vi "FlexMag - 24-03-2023.vi"() -> ()   [LabVIEW 2018] (continued)
                                n12774 = local read "ch4-3 transfer"() -> (w17942:bool)
                                n12775 = local read "ABORT"() -> (w17941:bool)
                                n12776 = Not(x=w17942) -> (.not. x?=w17940:bool)
                                n12777 = Compound Arithmetic op=OR(w17935, w17941, w17940) -> (w17939:bool)
                                }
                              }
                            }
                          }
                        }
                      }
                      frame True {
                      }
                    }
                  }
                }
              }
              frame #46 {
                n12778 = local read "ch4-3 transfer"() -> (w17949:bool)
                n12779 = case shown="True" w17949 {
                  frame False {
                  }
                  frame True {
                    n12780 = local read "ABORT"() -> (w17950:bool)
                    n12781 = case shown="False" w17950 {
                      frame False {
                        n12782 = local write "trns 4-3 led 22"(TRUE ("trns 1-2 led 1")) -> ()
                        n12783 = Wait (ms)(milliseconds to wait=u32 100) -> ()  [unwired: 1 out]
                      }
                      frame True {
                      }
                    }
                  }
                }
              }
              frame #47 {
                n12784 = local read "ch4-3 transfer"() -> (w17953:bool)
                n12785 = case shown="True" w17953 {
                  frame False {
                  }
                  frame True {
                    n12786 = local read "ABORT"() -> (w17954:bool)
                    n12787 = case shown="False" w17954 {
                      frame False {
                        n12788 = disable-structure shown="Enabled" {
                          frame Disabled {
                            n12789 = stacked-sequence {
                              frame #0 {
                                n12790 = while {
                                i -> [w17959]
                                stop <- w17960 stop-if-true
                                n12791 = Greater Or Equal?(x=w17959, y=100) -> (x >= y?=w17957:bool)
                                n12792 = case shown="True" w17957 {
                                frame False {
                                }
                                frame True {
                                n12793 = local write "Warning Message"("Transfer process canceled!\nRight Slow Sensor problem" ("Warning Message")) -> ()
                                n12794 = local write "trns error"(TRUE ("TRNS error")) -> ()
                                }
                                }
                                n12795 = local read "Cnt_Right_Slow DI"() -> (w17955:bool)
                                n12796 = case shown="True" w17955 {
                                tunnel: [TRUE ("CH1_Trns_BP_Left_DO") FALSE ("CH1_Trns_BP_Left_DO")] -> w17956
                                frame False {
                                }
                                frame True {
                                n12797 = Wait Until Next ms Multiple(millisecond multiple=u32 200) -> ()  [unwired: 1 out]
                                n12798 = local write "Cnt_Right_Slow DO"(FALSE ("TRNS error")) -> ()
                                }
                                }
                                n12799 = local read "ch4-3 transfer"() -> (w17963:bool)
                                n12800 = local read "ABORT"() -> (w17962:bool)
                                n12801 = Not(x=w17963) -> (.not. x?=w17961:bool)
                                n12802 = Compound Arithmetic op=OR(w17956, w17962, w17961) -> (w17960:bool)
                                }
                              }
                              frame #1 {
                                n12803 = while {
                                i -> [w17974]
                                stop <- w17975 stop-if-true
                                n12804 = Greater Or Equal?(x=w17974, y=100) -> (x >= y?=w17972:bool)
                                n12805 = case shown="True" w17972 {
                                frame False {
                                }
                                frame True {
                                n12806 = local write "Warning Message"("Transfer process canceled!\nRight Limit Sensor problem" ("Warning Message")) -> ()
                                n12807 = local write "trns error"(TRUE ("TRNS error")) -> ()
                                }
                                }
                                n12808 = local read "Cnt_Right_Limit DI"() -> (w17970:bool)
                                n12809 = case shown="True" w17970 {
                                tunnel: [TRUE ("CH1_Trns_BP_Left_DO") FALSE ("CH1_Trns_BP_Left_DO")] -> w17971
                                frame False {
                                }
                                frame True {
                                n12810 = Wait Until Next ms Multiple(millisecond multiple=u32 200) -> ()  [unwired: 1 out]
                                n12811 = local write "Cnt_Right_Limit DO"(FALSE ("TRNS error")) -> ()
                                }
                                }
                                n12812 = local read "ch4-3 transfer"() -> (w17978:bool)
                                n12813 = local read "ABORT"() -> (w17977:bool)
                                n12814 = Not(x=w17978) -> (.not. x?=w17976:bool)
                                n12815 = Compound Arithmetic op=OR(w17971, w17977, w17976) -> (w17975:bool)
                                }
                              }
                              frame #2 {
                                n12816 = while {
                                i -> [w17989]
                                stop <- w17990 stop-if-true
                                n12817 = Greater Or Equal?(x=w17989, y=100) -> (x >= y?=w17987:bool)
                                n12818 = case shown="True" w17987 {
                                frame False {
                                }
                                frame True {
                                n12819 = local write "Warning Message"("Transfer process canceled!\nLeft Slow Sensor problem" ("Warning Message")) -> ()
                                n12820 = local write "trns error"(TRUE ("TRNS error")) -> ()
                                }
                                }
                                n12821 = local read "Cnt_Left_Slow DI"() -> (w17985:bool)
                                n12822 = case shown="True" w17985 {
                                tunnel: [TRUE ("CH1_Trns_BP_Left_DO") FALSE ("CH1_Trns_BP_Left_DO")] -> w17986
                                frame False {
                                }
                                frame True {
                                n12823 = Wait Until Next ms Multiple(millisecond multiple=u32 200) -> ()  [unwired: 1 out]
                                n12824 = local write "Cnt_Left_Slow DO"(FALSE ("TRNS error")) -> ()
                                }
                                }
                                n12825 = local read "ch4-3 transfer"() -> (w17993:bool)
                                n12826 = local read "ABORT"() -> (w17992:bool)
                                n12827 = Not(x=w17993) -> (.not. x?=w17991:bool)
                                n12828 = Compound Arithmetic op=OR(w17986, w17992, w17991) -> (w17990:bool)
                                }
                              }
                              frame #3 {
                                n12829 = while {
                                i -> [w18004]
                                stop <- w18005 stop-if-true
                                n12830 = Greater Or Equal?(x=w18004, y=100) -> (x >= y?=w18002:bool)
                                n12831 = case shown="True" w18002 {
                                frame False {
                                }
                                frame True {
                                n12832 = local write "Warning Message"("Transfer process canceled!\nLeft Limit Sensor problem" ("Warning Message")) -> ()
                                n12833 = local write "trns error"(TRUE ("TRNS error")) -> ()
                                }
                                }
                                n12834 = local read "Cnt_Left_Limit DI"() -> (w18000:bool)
                                n12835 = case shown="True" w18000 {
                                tunnel: [TRUE ("CH1_Trns_BP_Left_DO") FALSE ("CH1_Trns_BP_Left_DO")] -> w18001
                                frame False {
                                }
                                frame True {
                                n12836 = Wait Until Next ms Multiple(millisecond multiple=u32 200) -> ()  [unwired: 1 out]
                                n12837 = local write "Cnt_Left_Limit DO"(FALSE ("TRNS error")) -> ()
                                }
                                }
                                n12838 = local read "ch4-3 transfer"() -> (w18008:bool)
                                n12839 = local read "ABORT"() -> (w18007:bool)
                                n12840 = Not(x=w18008) -> (.not. x?=w18006:bool)
                                n12841 = Compound Arithmetic op=OR(w18001, w18007, w18006) -> (w18005:bool)
                                }
                              }
                            }
                          }
                          frame Enabled {
                            w18016 = FALSE ("CH4_SRV1_Piston_For_DO")
                            w18017 = FALSE ("CH4_SRV1_Piston_For_DO")
                            n12842 = local write "CH1_Right_Limit_DO"(w18017) -> ()
                            n12843 = local write "CH1_Right_Slow_DO"(w18017) -> ()
                            n12844 = local write "CH2_Right_Limit_DO"(w18017) -> ()
                            n12845 = local write "CH2_Right_Slow_DO"(w18017) -> ()
                            n12846 = local write "CH2_Left_Slow_DO"(w18017) -> ()
                            n12847 = local write "CH2_Left_Limit_DO"(w18017) -> ()
                            n12848 = Wait (ms)(milliseconds to wait=u32 2000) -> ()  [unwired: 1 out]
                            n12849 = local write "CH3_Right_Limit_DO"(w18016) -> ()
                            n12850 = local write "CH3_Right_Slow_DO"(w18016) -> ()
                            n12851 = local write "CH3_Left_Slow_DO"(w18016) -> ()
                            n12852 = local write "CH3_Left_Limit_DO"(w18016) -> ()
                            n12853 = local write "CH4_Left_Limit_DO"(w18016) -> ()
                            n12854 = local write "CH4_Left_Slow_DO"(w18016) -> ()
                          }
                        }
                      }
                      frame True {
                      }
                    }
                  }
                }
              }
              frame #48 {
                n12855 = local read "ch4-3 transfer"() -> (w18018:bool)
                n12856 = case shown="True" w18018 {
                  frame False {
                  }
                  frame True {
                    n12857 = local read "ABORT"() -> (w18019:bool)
                    n12858 = case shown="False" w18019 {
                      frame False {
                        n12859 = local write "trns 4-3 led 23"(TRUE ("trns 1-2 led 17")) -> ()
                        n12860 = Wait (ms)(milliseconds to wait=u32 100) -> ()  [unwired: 1 out]
                      }
                      frame True {
                      }
                    }
                  }
                }
              }
              frame #49 {
                n12861 = local read "ch4-3 transfer"() -> (w18022:bool)
                n12862 = case shown="True" w18022 {
                  frame False {
                  }
                  frame True {
                    n12863 = local read "ABORT"() -> (w18023:bool)
                    n12864 = case shown="False" w18023 {
                      frame False {
                        n12865 = local write "Buzzer DO"(TRUE ("trns 1-2 led 17")) -> ()
                        n12866 = Wait (ms)(milliseconds to wait=u32 3000) -> ()  [unwired: 1 out]
                        n12867 = local write "System Status"("CH4 to CH3  Transfer Completed" ("System Status")) -> ()
                      }
                      frame True {
                      }
                    }
                  }
                }
              }
              frame #50 {
                n12868 = local read "ch4-3 transfer"() -> (w18027:bool)
                n12869 = case shown="True" w18027 {
                  frame False {
                  }
                  frame True {
                    n12870 = local read "ABORT"() -> (w18028:bool)
                    n12871 = case shown="False" w18028 {
                      frame False {
                        w18029 = u16 3 items=["CH1"=1, "CH2"=2, "CH3"=3, "CH4"=4] ("cassette position selection")
                        w18030 = FALSE ("trns 1-2 led 17")
                        n12872 = Wait (ms)(milliseconds to wait=u32 1000) -> ()  [unwired: 1 out]
                        n12873 = local write "ch4-3 transfer"(FALSE ("trns 1-2 led 17")) -> ()
                        n12874 = local write "Buzzer DO"(FALSE ("trns 1-2 led 17")) -> ()
                        n12875 = local write "cassette position selection"(w18029) -> ()
                        n12876 = local write "System Status"("SEMI-AUTOMATIC MODE " ("System Status")) -> ()
                        n12877 = Not(x=w18030) -> (.not. x?=w18031:bool)
                        n12878 = local write "present location"(3.0 ("present location")) -> ()
                        n12879 = local write "casette_ch1_gui"(w18030) -> ()
                        n12880 = local write "casette_ch2_gui"(w18030) -> ()
                        n12881 = local write "casette_ch3_gui"(w18031) -> ()
                        n12882 = local write "casette_ch4_gui"(w18030) -> ()
                      }
                      frame True {
                      }
                    }
                  }
                }
              }
              frame #51 {
              }
            }
          }
          frame True {
          }
        }
      }
    }
  }
  n12883 = while {
    stop <- FALSE stop-if-true
    n12884 = Wait Until Next ms Multiple(millisecond multiple=u32 300) -> ()  [unwired: 1 out]
    n12885 = case shown="True" "trns pre check" {
      frame False {
      }
      frame True {
        n12886 = stacked-sequence {
          frame #0 {
            n12887 = flat-sequence {
              frame #0 {
                n12888 = local write "trns clear"(TRUE ("trns clear")) -> ()
              }
              frame #1 {
                n12889 = Wait (ms)(milliseconds to wait=u32 1000) -> ()  [unwired: 1 out]
              }
            }
          }
          frame #1 {
            n12890 = local read "ABORT"() -> (w18042:bool)
            n12891 = case shown="False" w18042 {
              frame False {
                n12892 = local read "trns pre check"() -> (w18043:bool)
                n12893 = case shown="True" w18043 {
                  frame False {
                  }
                  frame True {
                    n12894 = while {
                      i -> [w18050]
                      stop <- w18047 stop-if-true
                      n12895 = Greater Or Equal?(x=w18050, y=600) -> (x >= y?=w18048:bool)
                      n12896 = case shown="True" w18048 {
                        frame False {
                        }
                        frame True {
                          n12897 = local write "Warning Message"("Transfer process canceled!\nCH1 srv piston problem" ("Warning Message")) -> ()
                          n12898 = local write "trns error"(TRUE ("TRNS error")) -> ()
                        }
                      }
                      n12899 = local read "CH1_SRV1_Piston_Back_DI"() -> (w18052:bool)
                      n12900 = case shown="True" w18052 {
                        tunnel: [FALSE TRUE] -> w18051
                        frame False {
                          n12901 = local write "CH1_SRV1_Piston_Back_DO"(TRUE ("CH1_SRV1_Piston_Back_DO")) -> ()
                          n12902 = local write "CH1_SRV1_Piston_For_DO"(FALSE ("CH1_SRV1_Piston_For_DO")) -> ()
                          n12903 = Wait Until Next ms Multiple(millisecond multiple=u32 200) -> ()  [unwired: 1 out]
                        }
                        frame True {
                        }
                      }
                      n12904 = local read "trns pre check"() -> (w18044:bool)
                      n12905 = local read "ABORT"() -> (w18046:bool)
                      n12906 = Not(x=w18044) -> (.not. x?=w18045:bool)
                      n12907 = Compound Arithmetic op=OR(w18051, w18046, w18045) -> (w18047:bool)
                    }
                  }
                }
              }
              frame True {
              }
            }
          }
          frame #2 {
            n12908 = local read "trns pre check"() -> (w18060:bool)
            n12909 = case shown="True" w18060 {
              frame False {
              }
              frame True {
                n12910 = local read "ABORT"() -> (w18061:bool)
                n12911 = case shown="False" w18061 {
                  frame False {
                    n12912 = local write "trns pre check led 1"(TRUE ("1")) -> ()
                    n12913 = Wait (ms)(milliseconds to wait=u32 100) -> ()  [unwired: 1 out]
                  }
                  frame True {
                  }
                }
              }
            }
          }
          frame #3 {
            n12914 = local read "ABORT"() -> (w18064:bool)
            n12915 = case shown="False" w18064 {
              frame False {
                n12916 = local read "trns pre check"() -> (w18065:bool)
                n12917 = case shown="True" w18065 {
                  frame False {
                  }
                  frame True {
                    n12918 = while {
                      i -> [w18072]
                      stop <- w18069 stop-if-true
                      n12919 = Greater Or Equal?(x=w18072, y=600) -> (x >= y?=w18070:bool)
                      n12920 = case shown="True" w18070 {
                        frame False {
                        }
                        frame True {
                          n12921 = local write "Warning Message"("Transfer process canceled!\nCH2 srv piston problem" ("Warning Message")) -> ()
                          n12922 = local write "trns error"(TRUE ("TRNS error")) -> ()
                        }
                      }
                      n12923 = local read "CH2_SRV1_Piston_Back_DI"() -> (w18074:bool)
                      n12924 = case shown="False" w18074 {
                        tunnel: [FALSE TRUE] -> w18073
                        frame False {
                          n12925 = local write "CH2_SRV1_Piston_Back_DO"(TRUE ("CH1_SRV1_Piston_Back_DO")) -> ()
                          n12926 = local write "CH2_SRV1_Piston_For_DO"(FALSE ("CH2_SRV1_Piston_For_DO")) -> ()
                          n12927 = Wait Until Next ms Multiple(millisecond multiple=u32 200) -> ()  [unwired: 1 out]
                        }
                        frame True {
                        }
                      }
                      n12928 = local read "trns pre check"() -> (w18066:bool)
                      n12929 = local read "ABORT"() -> (w18068:bool)
                      n12930 = Not(x=w18066) -> (.not. x?=w18067:bool)
                      n12931 = Compound Arithmetic op=OR(w18073, w18068, w18067) -> (w18069:bool)
                    }
                  }
                }
              }
              frame True {
              }
            }
          }
          frame #4 {
            n12932 = local read "trns pre check"() -> (w18082:bool)
            n12933 = case shown="True" w18082 {
              frame False {
              }
              frame True {
                n12934 = local read "ABORT"() -> (w18083:bool)
                n12935 = case shown="False" w18083 {
                  frame False {
                    n12936 = local write "trns pre check led 2"(TRUE ("1")) -> ()
                    n12937 = Wait (ms)(milliseconds to wait=u32 100) -> ()  [unwired: 1 out]
                  }
                  frame True {
                  }
                }
              }
            }
          }
          frame #5 {
            n12938 = local read "ABORT"() -> (w18086:bool)
            n12939 = case shown="False" w18086 {
              frame False {
                n12940 = local read "trns pre check"() -> (w18087:bool)
                n12941 = case shown="True" w18087 {
                  frame False {
                  }
                  frame True {
                    n12942 = while {
                      i -> [w18094]
                      stop <- w18091 stop-if-true
                      n12943 = Greater Or Equal?(x=w18094, y=600) -> (x >= y?=w18092:bool)
                      n12944 = case shown="True" w18092 {
                        frame False {
                        }
                        frame True {
                          n12945 = local write "Warning Message"("Transfer process canceled!\nCH3 srv piston problem" ("Warning Message")) -> ()
                          n12946 = local write "trns error"(TRUE ("TRNS error")) -> ()
                        }
                      }
                      n12947 = local read "CH3_SRV1_Piston_Back_DI"() -> (w18096:bool)
                      n12948 = case shown="False" w18096 {
                        tunnel: [FALSE TRUE] -> w18095
                        frame False {
                          n12949 = local write "CH3_SRV1_Piston_Back_DO"(TRUE ("CH1_SRV1_Piston_Back_DO")) -> ()
                          n12950 = local write "CH3_SRV1_Piston_For_DO"(FALSE ("CH3_SRV1_Piston_For_DO")) -> ()
                          n12951 = Wait Until Next ms Multiple(millisecond multiple=u32 200) -> ()  [unwired: 1 out]
                        }
                        frame True {
                        }
                      }
                      n12952 = local read "trns pre check"() -> (w18088:bool)
                      n12953 = local read "ABORT"() -> (w18090:bool)
                      n12954 = Not(x=w18088) -> (.not. x?=w18089:bool)
                      n12955 = Compound Arithmetic op=OR(w18095, w18090, w18089) -> (w18091:bool)
                    }
                  }
                }
              }
              frame True {
              }
            }
          }
          frame #6 {
            n12956 = local read "trns pre check"() -> (w18104:bool)
            n12957 = case shown="True" w18104 {
              frame False {
              }
              frame True {
                n12958 = local read "ABORT"() -> (w18105:bool)
                n12959 = case shown="False" w18105 {
                  frame False {
                    n12960 = local write "trns pre check led 3"(TRUE ("1")) -> ()
                    n12961 = Wait (ms)(milliseconds to wait=u32 100) -> ()  [unwired: 1 out]
                  }
                  frame True {
                  }
                }
              }
            }
          }
          frame #7 {
            n12962 = local read "ABORT"() -> (w18108:bool)
            n12963 = case shown="False" w18108 {
              frame False {
                n12964 = local read "trns pre check"() -> (w18109:bool)
                n12965 = case shown="True" w18109 {
                  frame False {
                  }
                  frame True {
                    n12966 = while {
                      i -> [w18116]
                      stop <- w18113 stop-if-true
                      n12967 = Greater Or Equal?(x=w18116, y=600) -> (x >= y?=w18114:bool)
                      n12968 = case shown="True" w18114 {
                        frame False {
                        }
                        frame True {
                          n12969 = local write "Warning Message"("Transfer process canceled!\nCH4 srv piston problem" ("Warning Message")) -> ()
                          n12970 = local write "trns error"(TRUE ("TRNS error")) -> ()
                        }
                      }
                      n12971 = local read "CH4_SRV1_Piston_Back_DI"() -> (w18118:bool)
                      n12972 = case shown="False" w18118 {
                        tunnel: [FALSE TRUE] -> w18117
                        frame False {
                          n12973 = local write "CH4_SRV1_Piston_Back_DO"(TRUE ("CH1_SRV1_Piston_Back_DO")) -> ()
                          n12974 = local write "CH4_SRV1_Piston_For_DO"(FALSE ("CH4_SRV1_Piston_For_DO")) -> ()
                          n12975 = Wait Until Next ms Multiple(millisecond multiple=u32 200) -> ()  [unwired: 1 out]
                        }
                        frame True {
                        }
                      }
                      n12976 = local read "trns pre check"() -> (w18110:bool)
                      n12977 = local read "ABORT"() -> (w18112:bool)
                      n12978 = Not(x=w18110) -> (.not. x?=w18111:bool)
                      n12979 = Compound Arithmetic op=OR(w18117, w18112, w18111) -> (w18113:bool)
                    }
                  }
                }
              }
              frame True {
              }
            }
          }
          frame #8 {
            n12980 = local read "trns pre check"() -> (w18126:bool)
            n12981 = case shown="True" w18126 {
              frame False {
              }
              frame True {
                n12982 = local read "ABORT"() -> (w18127:bool)
                n12983 = case shown="False" w18127 {
                  frame False {
                    n12984 = local write "trns pre check led 4"(TRUE ("1")) -> ()
                    n12985 = Wait (ms)(milliseconds to wait=u32 100) -> ()  [unwired: 1 out]
                  }
                  frame True {
                  }
                }
              }
            }
          }
          frame #9 {
            n12986 = local read "ABORT"() -> (w18130:bool)
            n12987 = case shown="False" w18130 {
              frame False {
                n12988 = local read "trns pre check"() -> (w18131:bool)
                n12989 = case shown="True" w18131 {
                  frame False {
                  }
                  frame True {
                    n12990 = while {
                      i -> [w18138]
                      stop <- w18135 stop-if-true
                      n12991 = Greater Or Equal?(x=w18138, y=600) -> (x >= y?=w18136:bool)
                      n12992 = case shown="True" w18136 {
                        frame False {
                        }
                        frame True {
                          n12993 = local write "Warning Message"("Transfer process canceled!\nCH1 PetCool problem" ("Warning Message")) -> ()
                          n12994 = local write "trns error"(TRUE ("TRNS error")) -> ()
                        }
                      }
                      n12995 = local read "CH1_PetCool_Up_DI"() -> (w18140:bool)
                      n12996 = case shown="False" w18140 {
                        tunnel: [FALSE TRUE] -> w18139
                        frame False {
                          n12997 = local write "CH1_PetCool_Down_DO"(FALSE ("CH4_SRV1_Piston_For_DO")) -> ()
                          n12998 = local write "CH1_PetCool_Up_DO"(TRUE ("CH1_SRV1_Piston_Back_DO")) -> ()
                          n12999 = Wait Until Next ms Multiple(millisecond multiple=u32 200) -> ()  [unwired: 1 out]
                        }
                        frame True {
                        }
                      }
                      n13000 = local read "trns pre check"() -> (w18132:bool)
                      n13001 = local read "ABORT"() -> (w18134:bool)
                      n13002 = Not(x=w18132) -> (.not. x?=w18133:bool)
                      n13003 = Compound Arithmetic op=OR(w18139, w18134, w18133) -> (w18135:bool)
                    }
                  }
                }
              }
              frame True {
              }
            }
          }
          frame #10 {
            n13004 = local read "trns pre check"() -> (w18148:bool)
            n13005 = case shown="True" w18148 {
              frame False {
              }
              frame True {
                n13006 = local read "ABORT"() -> (w18149:bool)
                n13007 = case shown="False" w18149 {
                  frame False {
                    n13008 = local write "trns pre check led 5"(TRUE ("1")) -> ()
                    n13009 = Wait (ms)(milliseconds to wait=u32 100) -> ()  [unwired: 1 out]
                  }
                  frame True {
                  }
                }
              }
            }
          }
          frame #11 {
            n13010 = local read "ABORT"() -> (w18152:bool)
            n13011 = case shown="False" w18152 {
              frame False {
                n13012 = local read "trns pre check"() -> (w18153:bool)
                n13013 = case shown="True" w18153 {
                  frame False {
                  }
                  frame True {
                    n13014 = while {
                      i -> [w18160]
                      stop <- w18157 stop-if-true
                      n13015 = Greater Or Equal?(x=w18160, y=600) -> (x >= y?=w18158:bool)
                      n13016 = case shown="True" w18158 {
                        frame False {
                        }
                        frame True {
                          n13017 = local write "Warning Message"("Transfer process canceled!\nCH2 PetCool problem" ("Warning Message")) -> ()
                          n13018 = local write "trns error"(TRUE ("TRNS error")) -> ()
                        }
                      }
                      n13019 = local read "CH2_PetCool_Up_DI"() -> (w18162:bool)
                      n13020 = case shown="False" w18162 {
                        tunnel: [FALSE TRUE] -> w18161
                        frame False {
                          n13021 = local write "CH2_PetCool_Down_DO"(FALSE ("CH4_SRV1_Piston_For_DO")) -> ()
                          n13022 = local write "CH2_PetCool_Up_DO"(TRUE ("CH1_SRV1_Piston_Back_DO")) -> ()
                          n13023 = Wait Until Next ms Multiple(millisecond multiple=u32 200) -> ()  [unwired: 1 out]
                        }
                        frame True {
                        }
                      }
                      n13024 = local read "trns pre check"() -> (w18154:bool)
                      n13025 = local read "ABORT"() -> (w18156:bool)
                      n13026 = Not(x=w18154) -> (.not. x?=w18155:bool)
                      n13027 = Compound Arithmetic op=OR(w18161, w18156, w18155) -> (w18157:bool)
                    }
                  }
                }
              }
              frame True {
              }
            }
          }
          frame #12 {
            n13028 = local read "trns pre check"() -> (w18170:bool)
            n13029 = case shown="True" w18170 {
              frame False {
              }
              frame True {
                n13030 = local read "ABORT"() -> (w18171:bool)
                n13031 = case shown="False" w18171 {
                  frame False {
                    n13032 = local write "trns pre check led 6"(TRUE ("1")) -> ()
                    n13033 = Wait (ms)(milliseconds to wait=u32 100) -> ()  [unwired: 1 out]
                  }
                  frame True {
                  }
                }
              }
            }
          }
          frame #13 {
            n13034 = local read "ABORT"() -> (w18174:bool)
            n13035 = case shown="False" w18174 {
              frame False {
                n13036 = local read "trns pre check"() -> (w18175:bool)
                n13037 = case shown="True" w18175 {
                  frame False {
                  }
                  frame True {
                    n13038 = while {
                      i -> [w18182]
                      stop <- w18179 stop-if-true
                      n13039 = Greater Or Equal?(x=w18182, y=600) -> (x >= y?=w18180:bool)
                      n13040 = case shown="True" w18180 {
                        frame False {
                        }
                        frame True {
                          n13041 = local write "Warning Message"("Transfer process canceled!\nCH3 PetCool problem" ("Warning Message")) -> ()
                          n13042 = local write "trns error"(TRUE ("TRNS error")) -> ()
                        }
                      }
                      n13043 = local read "CH3_PetCool_Up_DI"() -> (w18184:bool)
                      n13044 = case shown="False" w18184 {
                        tunnel: [FALSE TRUE] -> w18183
                        frame False {
                          n13045 = local write "CH3_PetCool_Down_DO"(FALSE ("CH4_SRV1_Piston_For_DO")) -> ()
                          n13046 = local write "CH3_PetCool_Up_DO"(TRUE ("CH1_SRV1_Piston_Back_DO")) -> ()
                          n13047 = Wait Until Next ms Multiple(millisecond multiple=u32 200) -> ()  [unwired: 1 out]
                        }
                        frame True {
                        }
                      }
                      n13048 = local read "trns pre check"() -> (w18176:bool)
                      n13049 = local read "ABORT"() -> (w18178:bool)
                      n13050 = Not(x=w18176) -> (.not. x?=w18177:bool)
                      n13051 = Compound Arithmetic op=OR(w18183, w18178, w18177) -> (w18179:bool)
                    }
                  }
                }
              }
              frame True {
              }
            }
          }
          frame #14 {
            n13052 = local read "trns pre check"() -> (w18192:bool)
            n13053 = case shown="True" w18192 {
              frame False {
              }
              frame True {
                n13054 = local read "ABORT"() -> (w18193:bool)
                n13055 = case shown="False" w18193 {
                  frame False {
                    n13056 = local write "trns pre check led 7"(TRUE ("1")) -> ()
                    n13057 = Wait (ms)(milliseconds to wait=u32 100) -> ()  [unwired: 1 out]
                  }
                  frame True {
                  }
                }
              }
            }
          }
          frame #15 {
            n13058 = local read "ABORT"() -> (w18196:bool)
            n13059 = case shown="False" w18196 {
              frame False {
                n13060 = local read "trns pre check"() -> (w18197:bool)
                n13061 = case shown="True" w18197 {
                  frame False {
                  }
                  frame True {
                    n13062 = while {
                      i -> [w18204]
                      stop <- w18201 stop-if-true
                      n13063 = Greater Or Equal?(x=w18204, y=600) -> (x >= y?=w18202:bool)
                      n13064 = case shown="True" w18202 {
                        frame False {
                        }
                        frame True {
                          n13065 = local write "Warning Message"("Transfer process canceled!\nCH4 PetCool problem" ("Warning Message")) -> ()
                          n13066 = local write "trns error"(TRUE ("TRNS error")) -> ()
                        }
                      }
                      n13067 = local read "CH4_PetCool_Up_DI"() -> (w18206:bool)
                      n13068 = case shown="False" w18206 {
                        tunnel: [FALSE TRUE] -> w18205
                        frame False {
                          n13069 = local write "CH4_PetCool_Down_DO"(FALSE ("CH4_SRV1_Piston_For_DO")) -> ()
                          n13070 = local write "CH4_PetCool_Up_DO"(TRUE ("CH1_SRV1_Piston_Back_DO")) -> ()
                          n13071 = Wait Until Next ms Multiple(millisecond multiple=u32 200) -> ()  [unwired: 1 out]
                        }
                        frame True {
                        }
                      }
                      n13072 = local read "trns pre check"() -> (w18198:bool)
                      n13073 = local read "ABORT"() -> (w18200:bool)
                      n13074 = Not(x=w18198) -> (.not. x?=w18199:bool)
                      n13075 = Compound Arithmetic op=OR(w18205, w18200, w18199) -> (w18201:bool)
                    }
                  }
                }
              }
              frame True {
              }
            }
          }
          frame #16 {
            n13076 = local read "trns pre check"() -> (w18214:bool)
            n13077 = case shown="True" w18214 {
              frame False {
              }
              frame True {
                n13078 = local read "ABORT"() -> (w18215:bool)
                n13079 = case shown="False" w18215 {
                  frame False {
                    n13080 = local write "trns pre check led 8"(TRUE ("1")) -> ()
                    n13081 = Wait (ms)(milliseconds to wait=u32 100) -> ()  [unwired: 1 out]
                  }
                  frame True {
                  }
                }
              }
            }
          }
          frame #17 {
            n13082 = local read "ABORT"() -> (w18218:bool)
            n13083 = case shown="False" w18218 {
              frame False {
                n13084 = local read "trns pre check"() -> (w18219:bool)
                n13085 = case shown="True" w18219 {
                  frame False {
                  }
                  frame True {
                    n13086 = while {
                      i -> [w18226]
                      stop <- w18223 stop-if-true
                      n13087 = Greater Or Equal?(x=w18226, y=600) -> (x >= y?=w18224:bool)
                      n13088 = case shown="True" w18224 {
                        frame False {
                        }
                        frame True {
                          n13089 = local write "Warning Message"("Transfer process canceled!\nCH1 Cassette Fix problem" ("Warning Message")) -> ()
                          n13090 = local write "trns error"(TRUE ("TRNS error")) -> ()
                        }
                      }
                      n13091 = local read "CH1_Cst_Fix_Up_DI"() -> (w18228:bool)
                      n13092 = case shown="False" w18228 {
                        tunnel: [FALSE TRUE] -> w18227
                        frame False {
                          n13093 = local write "CH1_Cst_Fix_DO"(FALSE ("CH1_SRV1_Piston_Back_DO")) -> ()
                          n13094 = Wait Until Next ms Multiple(millisecond multiple=u32 200) -> ()  [unwired: 1 out]
                        }
                        frame True {
                        }
                      }
                      n13095 = local read "trns pre check"() -> (w18220:bool)
                      n13096 = local read "ABORT"() -> (w18222:bool)
                      n13097 = Not(x=w18220) -> (.not. x?=w18221:bool)
                      n13098 = Compound Arithmetic op=OR(w18227, w18222, w18221) -> (w18223:bool)
                    }
                  }
                }
              }
              frame True {
              }
            }
          }
          frame #18 {
            n13099 = local read "trns pre check"() -> (w18235:bool)
            n13100 = case shown="True" w18235 {
              frame False {
              }
              frame True {
                n13101 = local read "ABORT"() -> (w18236:bool)
                n13102 = case shown="False" w18236 {
                  frame False {
                    n13103 = local write "trns pre check led 9"(TRUE ("1")) -> ()
                    n13104 = Wait (ms)(milliseconds to wait=u32 100) -> ()  [unwired: 1 out]
                  }
                  frame True {
                  }
                }
              }
            }
          }
          frame #19 {
            n13105 = local read "ABORT"() -> (w18239:bool)
            n13106 = case shown="False" w18239 {
              frame False {
                n13107 = local read "trns pre check"() -> (w18240:bool)
                n13108 = case shown="True" w18240 {
                  frame False {
                  }
                  frame True {
                    n13109 = while {
                      i -> [w18247]
                      stop <- w18244 stop-if-true
                      n13110 = Greater Or Equal?(x=w18247, y=600) -> (x >= y?=w18245:bool)
                      n13111 = case shown="True" w18245 {
                        frame False {
                        }
                        frame True {
                          n13112 = local write "Warning Message"("Transfer process canceled!\nCH2 Cassette Fix problem" ("Warning Message")) -> ()
                          n13113 = local write "trns error"(TRUE ("TRNS error")) -> ()
                        }
                      }
                      n13114 = local read "CH2_Cst_Fix_Up_DI"() -> (w18249:bool)
                      n13115 = case shown="False" w18249 {
                        tunnel: [FALSE TRUE] -> w18248
                        frame False {
                          n13116 = local write "CH2_Cst_Fix_DO"(FALSE ("CH1_SRV1_Piston_Back_DO")) -> ()
                          n13117 = Wait Until Next ms Multiple(millisecond multiple=u32 200) -> ()  [unwired: 1 out]
                        }
                        frame True {
                        }
                      }
                      n13118 = local read "trns pre check"() -> (w18241:bool)
                      n13119 = local read "ABORT"() -> (w18243:bool)
                      n13120 = Not(x=w18241) -> (.not. x?=w18242:bool)
                      n13121 = Compound Arithmetic op=OR(w18248, w18243, w18242) -> (w18244:bool)
                    }
                  }
                }
              }
              frame True {
              }
            }
          }
          frame #20 {
            n13122 = local read "trns pre check"() -> (w18256:bool)
            n13123 = case shown="True" w18256 {
              frame False {
              }
              frame True {
                n13124 = local read "ABORT"() -> (w18257:bool)
                n13125 = case shown="False" w18257 {
                  frame False {
                    n13126 = local write "trns pre check led 10"(TRUE ("1")) -> ()
                    n13127 = Wait (ms)(milliseconds to wait=u32 100) -> ()  [unwired: 1 out]
                  }
                  frame True {
                  }
                }
              }
            }
          }
          frame #21 {
            n13128 = local read "ABORT"() -> (w18260:bool)
            n13129 = case shown="False" w18260 {
              frame False {
                n13130 = local read "trns pre check"() -> (w18261:bool)
                n13131 = case shown="True" w18261 {
                  frame False {
                  }
                  frame True {
                    n13132 = while {
                      i -> [w18268]
                      stop <- w18265 stop-if-true
                      n13133 = Greater Or Equal?(x=w18268, y=600) -> (x >= y?=w18266:bool)
                      n13134 = case shown="True" w18266 {
                        frame False {
                        }
                        frame True {
                          n13135 = local write "Warning Message"("Transfer process canceled!\nCH3 Cassette Fix problem" ("Warning Message")) -> ()
                          n13136 = local write "trns error"(TRUE ("TRNS error")) -> ()
                        }
                      }
                      n13137 = local read "CH3_Cst_Fix_Up_DI"() -> (w18270:bool)
                      n13138 = case shown="False" w18270 {
                        tunnel: [FALSE TRUE] -> w18269
                        frame False {
                          n13139 = local write "CH3_Cst_Fix_DO"(FALSE ("CH1_SRV1_Piston_Back_DO")) -> ()
                          n13140 = Wait Until Next ms Multiple(millisecond multiple=u32 200) -> ()  [unwired: 1 out]
                        }
                        frame True {
                        }
                      }
                      n13141 = local read "trns pre check"() -> (w18262:bool)
                      n13142 = local read "ABORT"() -> (w18264:bool)
                      n13143 = Not(x=w18262) -> (.not. x?=w18263:bool)
                      n13144 = Compound Arithmetic op=OR(w18269, w18264, w18263) -> (w18265:bool)
                    }
                  }
                }
              }
              frame True {
              }
            }
          }
          frame #22 {
            n13145 = local read "trns pre check"() -> (w18277:bool)
            n13146 = case shown="True" w18277 {
              frame False {
              }
              frame True {
                n13147 = local read "ABORT"() -> (w18278:bool)
                n13148 = case shown="False" w18278 {
                  frame False {
                    n13149 = local write "trns pre check led 11"(TRUE ("1")) -> ()
                    n13150 = Wait (ms)(milliseconds to wait=u32 100) -> ()  [unwired: 1 out]
                  }
                  frame True {
                  }
                }
              }
            }
          }
          frame #23 {
            n13151 = local read "ABORT"() -> (w18281:bool)
            n13152 = case shown="False" w18281 {
              frame False {
                n13153 = local read "trns pre check"() -> (w18282:bool)
                n13154 = case shown="True" w18282 {
                  frame False {
                  }
                  frame True {
                    n13155 = while {
                      i -> [w18289]
                      stop <- w18286 stop-if-true
                      n13156 = Greater Or Equal?(x=w18289, y=600) -> (x >= y?=w18287:bool)
                      n13157 = case shown="True" w18287 {
                        frame False {
                        }
                        frame True {
                          n13158 = local write "Warning Message"("Transfer process canceled!\nCH4 Cassette Fix problem" ("Warning Message")) -> ()
                          n13159 = local write "trns error"(TRUE ("TRNS error")) -> ()
                        }
                      }
                      n13160 = local read "CH4_Cst_Fix_Up_DI"() -> (w18291:bool)
                      n13161 = case shown="False" w18291 {
                        tunnel: [FALSE TRUE] -> w18290
                        frame False {
                          n13162 = local write "CH4_Cst_Fix_DO"(FALSE ("CH1_SRV1_Piston_Back_DO")) -> ()
                          n13163 = Wait Until Next ms Multiple(millisecond multiple=u32 200) -> ()  [unwired: 1 out]
                        }
                        frame True {
                        }
                      }
                      n13164 = local read "trns pre check"() -> (w18283:bool)
                      n13165 = local read "ABORT"() -> (w18285:bool)
                      n13166 = Not(x=w18283) -> (.not. x?=w18284:bool)
                      n13167 = Compound Arithmetic op=OR(w18290, w18285, w18284) -> (w18286:bool)
                    }
                  }
                }
              }
              frame True {
              }
            }
          }
          frame #24 {
            n13168 = local read "trns pre check"() -> (w18298:bool)
            n13169 = case shown="True" w18298 {
              frame False {
              }
              frame True {
                n13170 = local read "ABORT"() -> (w18299:bool)
                n13171 = case shown="False" w18299 {
                  frame False {
                    n13172 = local write "trns pre check led 12"(TRUE ("1")) -> ()
                    n13173 = Wait (ms)(milliseconds to wait=u32 100) -> ()  [unwired: 1 out]
                  }
                  frame True {
                  }
                }
              }
            }
          }
          frame #25 {
            n13174 = local read "trns pre check"() -> (w18302:bool)
            n13175 = case shown="True" w18302 {
              frame False {
              }
              frame True {
                n13176 = local read "ABORT"() -> (w18303:bool)
                n13177 = case shown="False" w18303 {
                  frame False {
                    n13178 = local write "trns pre check"(FALSE ("trns pre check")) -> ()
                    n13179 = Wait (ms)(milliseconds to wait=u32 100) -> ()  [unwired: 1 out]
                  }
                  frame True {
                  }
                }
              }
            }
          }
        }
      }
    }
  }
  n13180 = while {
    stop <- FALSE stop-if-true
    n13181 = local read "ABORT"() -> (w18307:bool)
    n13182 = Wait Until Next ms Multiple(millisecond multiple=u32 300) -> ()  [unwired: 1 out]
    n13183 = case shown="True" "TC parameter set" {
      tunnel: w18307 -> [_ w18314]
      tunnel: "Roll Forw" -> [_ w18313]
      frame False {
        "parameters led" <- FALSE
      }
      frame True {
        n13184 = case shown="False" w18314 {
          tunnel: w18313 -> [w18315 _]
          frame False {
            n13185 = case shown="True" w18315 {
              frame False {
                n13186 = stacked-sequence {
                  frame #0 {
                    n13187 = local write "TC1_close_loop_coefficient"(sgl 0.0 ("TC1_close_loop_coefficient")) -> ()
                    n13188 = local write "TC1_speed_coefficient_value"(sgl 100.0 ("TC1_speed_coefficient_value")) -> ()
                    n13189 = local write "TC1_AO1_upper_limit_value"(sgl 10.0 ("TC1_speed_coefficient_value")) -> ()
                    n13190 = local write "TC1_regulation_type_value"(sgl 0.0 ("TC1_speed_coefficient_value")) -> ()
                    n13191 = local write "TC1_AO1_bottom_limit_value"(sgl 0.0 ("TC1_speed_coefficient_value")) -> ()
                    n13192 = local write "TC1_setpoint_type_value"(sgl 0.0 ("TC1_speed_coefficient_value")) -> ()
                    n13193 = Wait (ms)(milliseconds to wait=u32 100) -> ()  [unwired: 1 out]
                    n13194 = local write "TC1_speed_gain_value"(sgl 0.0 ("TC1_speed_gain_value")) -> ()
                    n13195 = local write "TC2_close_loop_coefficient"(sgl 100.0 ("TC2_close_loop_coefficient")) -> ()
                    n13196 = local write "TC2_speed_coefficient_value"(sgl 0.0 ("TC2_speed_coefficient_value")) -> ()
                    n13197 = local write "TC2_AO1_upper_limit_value"(sgl 10.0 ("TC2_speed_gain_value")) -> ()
                    n13198 = local write "TC2_regulation_type_value"(sgl 1.0 ("TC2_speed_coefficient_value")) -> ()
                    n13199 = local write "TC2_speed_gain_value"(sgl 0.0 ("TC2_speed_gain_value")) -> ()
                    n13200 = local write "TC2_AO1_bottom_limit_value"(sgl 0.0 ("TC2_speed_coefficient_value")) -> ()
                    n13201 = local write "TC2_setpoint_type_value"(sgl 0.0 ("TC2_speed_coefficient_value")) -> ()
                  }
                  frame #1 {
                    n13202 = local write "TC1_close_loop_set"(TRUE ("TC1_close_loop_set")) -> ()
                  }
                  frame #2 {
                    n13203 = flat-sequence {
                      frame #0 {
                        n13204 = local read "waiting_TC"() -> (w18332:u32)
                        n13205 = Wait (ms)(milliseconds to wait=w18332) -> ()  [unwired: 1 out]
                      }
                      frame #1 {
                        n13206 = while {
                          stop <- w18333 stop-if-true
                          n13207 = local read "TC1_close_loop_set"() -> (w18334:bool)
                          n13208 = Wait Until Next ms Multiple(millisecond multiple=u32 300) -> ()  [unwired: 1 out]
                          n13209 = Not(x=w18334) -> (.not. x?=w18333:bool)
                        }
                      }
                    }
                  }
                  frame #3 {
                    n13210 = local write "TC1_speed_gain_set"(TRUE ("TC1_close_loop_set")) -> ()
                  }
                  frame #4 {
                    n13211 = flat-sequence {
                      frame #0 {
                        n13212 = local read "waiting_TC"() -> (w18337:u32)
                        n13213 = Wait (ms)(milliseconds to wait=w18337) -> ()  [unwired: 1 out]
                      }
                      frame #1 {
                        n13214 = while {
                          stop <- w18339 stop-if-true
                          n13215 = local read "TC1_speed_gain_set"() -> (w18338:bool)
                          n13216 = Wait Until Next ms Multiple(millisecond multiple=u32 300) -> ()  [unwired: 1 out]
                          n13217 = Not(x=w18338) -> (.not. x?=w18339:bool)
                        }
                      }
                    }
                  }
                  frame #5 {
                    n13218 = local write "TC1_speed_coefficient_set"(TRUE ("TC1_close_loop_set")) -> ()
                  }
                  frame #6 {
                    n13219 = flat-sequence {
                      frame #0 {
                        n13220 = local read "waiting_TC"() -> (w18342:u32)
                        n13221 = Wait (ms)(milliseconds to wait=w18342) -> ()  [unwired: 1 out]
                      }
                      frame #1 {
                        n13222 = while {
                          stop <- w18343 stop-if-true
                          n13223 = local read "TC1_speed_coefficient_set"() -> (w18344:bool)
                          n13224 = Wait Until Next ms Multiple(millisecond multiple=u32 300) -> ()  [unwired: 1 out]
                          n13225 = Not(x=w18344) -> (.not. x?=w18343:bool)
                        }
                      }
                    }
                  }
                  frame #7 {
                    n13226 = local write "TC1_AO1_polarity(neg_to_pos)"(TRUE ("TC1_close_loop_set")) -> ()
                  }
                  frame #8 {
                    n13227 = flat-sequence {
                      frame #0 {
                        n13228 = local read "waiting_TC"() -> (w18347:u32)
                        n13229 = Wait (ms)(milliseconds to wait=w18347) -> ()  [unwired: 1 out]
                      }
                      frame #1 {
                        n13230 = while {
                          stop <- w18349 stop-if-true
                          n13231 = local read "TC1_AO1_polarity(neg_to_pos)"() -> (w18348:bool)
                          n13232 = Wait Until Next ms Multiple(millisecond multiple=u32 300) -> ()  [unwired: 1 out]
                          n13233 = Not(x=w18348) -> (.not. x?=w18349:bool)
                        }
                      }
                    }
                  }
                  frame #9 {
                    n13234 = local write "TC2_close_loop_set"(TRUE ("TC1_close_loop_set")) -> ()
                  }
                  frame #10 {
                    n13235 = flat-sequence {
                      frame #0 {
                        n13236 = local read "waiting_TC"() -> (w18352:u32)
                        n13237 = Wait (ms)(milliseconds to wait=w18352) -> ()  [unwired: 1 out]
                      }
                      frame #1 {
                        n13238 = while {
                          stop <- w18353 stop-if-true
                          n13239 = local read "TC2_close_loop_set"() -> (w18354:bool)
                          n13240 = Wait Until Next ms Multiple(millisecond multiple=u32 300) -> ()  [unwired: 1 out]
                          n13241 = Not(x=w18354) -> (.not. x?=w18353:bool)
                        }
                      }
                    }
                  }
                  frame #11 {
                    n13242 = local write "TC2_speed_gain_set"(TRUE ("TC1_close_loop_set")) -> ()
                  }
                  frame #12 {
                    n13243 = flat-sequence {
                      frame #0 {
                        n13244 = local read "waiting_TC"() -> (w18357:u32)
                        n13245 = Wait (ms)(milliseconds to wait=w18357) -> ()  [unwired: 1 out]
                      }
                      frame #1 {
                        n13246 = while {
                          stop <- w18359 stop-if-true
                          n13247 = local read "TC2_speed_gain_set"() -> (w18358:bool)
                          n13248 = Wait Until Next ms Multiple(millisecond multiple=u32 300) -> ()  [unwired: 1 out]